vi "FlexMag - 23-03-2023.vi"() -> ()   [LabVIEW 2018] (continued)
                            }
                          }
                          n8986 = local read "CH3_Trns_BP_Right_DI"() -> (w14489:bool)
                          n8987 = case shown="False" w14489 {
                            tunnel: [FALSE ("CH1_Trns_BP_Left_DO") TRUE ("CH1_Trns_BP_Left_DO")] -> w14488
                            frame False {
                              n8988 = Wait Until Next ms Multiple(millisecond multiple=u32 200) -> ()  [unwired: 1 out]
                              n8989 = local write "CH3_Trns_BP_Right_DO"(TRUE ("CH1_Trns_BP_Left_DO")) -> ()
                            }
                            frame True {
                            }
                          }
                          n8990 = local read "ch2-3 transfer"() -> (w14496:bool)
                          n8991 = local read "ABORT"() -> (w14495:bool)
                          n8992 = Not(x=w14496) -> (.not. x?=w14494:bool)
                          n8993 = Compound Arithmetic op=OR(w14488, w14495, w14494) -> (w14493:bool)
                        }
                      }
                      frame True {
                      }
                    }
                  }
                }
              }
              frame #6 {
                n8994 = local read "ch2-3 transfer"() -> (w14503:bool)
                n8995 = case shown="True" w14503 {
                  frame False {
                  }
                  frame True {
                    n8996 = local read "ABORT"() -> (w14504:bool)
                    n8997 = case shown="False" w14504 {
                      frame False {
                        n8998 = local write "trns 2-3 led 2"(TRUE ("trns 1-2 led 1")) -> ()
                        n8999 = Wait (ms)(milliseconds to wait=u32 100) -> ()  [unwired: 1 out]
                      }
                      frame True {
                      }
                    }
                  }
                }
              }
              frame #7 {
                n9000 = local read "ch2-3 transfer"() -> (w14507:bool)
                n9001 = case shown="True" w14507 {
                  frame False {
                  }
                  frame True {
                    n9002 = local read "ABORT"() -> (w14508:bool)
                    n9003 = case shown="False" w14508 {
                      frame False {
                        n9004 = stacked-sequence {
                          frame #0 {
                            n9005 = local write "CH2_Trns_GV_Close_DO"(FALSE ("CH1_Trns_Gv_Close_DO")) -> ()
                            n9006 = Wait (ms)(milliseconds to wait=u32 100) -> ()  [unwired: 1 out]
                          }
                          frame #1 {
                            n9007 = while {
                              i -> [w14515]
                              stop <- w14516 stop-if-true
                              n9008 = Greater Or Equal?(x=w14515, y=600) -> (x >= y?=w14513:bool)
                              n9009 = case shown="True" w14513 {
                                frame False {
                                }
                                frame True {
                                n9010 = local write "trns error"(TRUE ("TRNS error")) -> ()
                                n9011 = local write "Warning Message"("Transfer process canceled!\nCH2-CH3 Trns GV couln't be opened" ("Warning Message")) -> ()
                                }
                              }
                              n9012 = local read "CH2_Trns_Gv_Open_DI"() -> (w14512:bool)
                              n9013 = case shown="False" w14512 {
                                tunnel: [FALSE ("CH1_Trns_BP_Left_DO") TRUE ("CH1_Trns_BP_Left_DO")] -> w14511
                                frame False {
                                n9014 = local write "CH2_Trns_GV_Open_DO"(TRUE ("CH1_Trns_BP_Left_DO")) -> ()
                                n9015 = Wait Until Next ms Multiple(millisecond multiple=u32 200) -> ()  [unwired: 1 out]
                                }
                                frame True {
                                }
                              }
                              n9016 = local read "ch2-3 transfer"() -> (w14519:bool)
                              n9017 = local read "ABORT"() -> (w14518:bool)
                              n9018 = Not(x=w14519) -> (.not. x?=w14517:bool)
                              n9019 = Compound Arithmetic op=OR(w14511, w14518, w14517) -> (w14516:bool)
                            }
                          }
                        }
                      }
                      frame True {
                      }
                    }
                  }
                }
              }
              frame #8 {
                n9020 = local read "ch2-3 transfer"() -> (w14526:bool)
                n9021 = case shown="True" w14526 {
                  frame False {
                  }
                  frame True {
                    n9022 = local read "ABORT"() -> (w14527:bool)
                    n9023 = case shown="False" w14527 {
                      frame False {
                        n9024 = local write "trns 2-3 led 3"(TRUE ("trns 1-2 led 1")) -> ()
                        n9025 = Wait (ms)(milliseconds to wait=u32 100) -> ()  [unwired: 1 out]
                      }
                      frame True {
                      }
                    }
                  }
                }
              }
              frame #9 {
                n9026 = local read "ch2-3 transfer"() -> (w14530:bool)
                n9027 = case shown="True" w14530 {
                  frame False {
                  }
                  frame True {
                    n9028 = local read "ABORT"() -> (w14531:bool)
                    n9029 = case shown="False" w14531 {
                      frame False {
                        n9030 = while {
                          i -> [w14536]
                          stop <- w14537 stop-if-true
                          n9031 = Greater Or Equal?(x=w14536, y=100) -> (x >= y?=w14534:bool)
                          n9032 = case shown="True" w14534 {
                            frame False {
                            }
                            frame True {
                              n9033 = local write "trns error"(TRUE ("TRNS error")) -> ()
                              n9034 = local write "Warning Message"("Transfer process canceled!\nCH2 TGV Control Problem" ("Warning Message")) -> ()
                            }
                          }
                          n9035 = local read "CH2_TGV_Control_DI"() -> (w14533:bool)
                          n9036 = case shown="True" w14533 {
                            tunnel: [TRUE ("CH1_Trns_BP_Left_DO") FALSE ("CH1_Trns_BP_Left_DO")] -> w14532
                            frame False {
                            }
                            frame True {
                              n9037 = Wait Until Next ms Multiple(millisecond multiple=u32 200) -> ()  [unwired: 1 out]
                              n9038 = local write "CH2_TGV_Control_DO"(FALSE ("CH1_Trns_BP_Left_DO")) -> ()
                            }
                          }
                          n9039 = local read "ch2-3 transfer"() -> (w14540:bool)
                          n9040 = local read "ABORT"() -> (w14539:bool)
                          n9041 = Not(x=w14540) -> (.not. x?=w14538:bool)
                          n9042 = Compound Arithmetic op=OR(w14532, w14539, w14538) -> (w14537:bool)
                        }
                      }
                      frame True {
                      }
                    }
                  }
                }
              }
              frame #10 {
                n9043 = local read "ch2-3 transfer"() -> (w14547:bool)
                n9044 = case shown="True" w14547 {
                  frame False {
                  }
                  frame True {
                    n9045 = local read "ABORT"() -> (w14548:bool)
                    n9046 = case shown="False" w14548 {
                      frame False {
                        n9047 = local write "trns 2-3 led 4"(TRUE ("trns 1-2 led 1")) -> ()
                        n9048 = Wait (ms)(milliseconds to wait=u32 100) -> ()  [unwired: 1 out]
                      }
                      frame True {
                      }
                    }
                  }
                }
              }
              frame #11 {
                n9049 = local read "ch2-3 transfer"() -> (w14551:bool)
                n9050 = case shown="True" w14551 {
                  frame False {
                  }
                  frame True {
                    n9051 = local read "ABORT"() -> (w14552:bool)
                    n9052 = case shown="False" w14552 {
                      frame False {
                        n9053 = while {
                          i -> [w14557]
                          stop <- w14558 stop-if-true
                          n9054 = local read "CH1_Trns_Interlock_DI"() -> (w14553:bool)
                          n9055 = Greater Or Equal?(x=w14557, y=100) -> (x >= y?=w14555:bool)
                          n9056 = case shown="True" w14555 {
                            frame False {
                            }
                            frame True {
                              n9057 = local write "Warning Message"("Transfer process canceled!\nCH1 Interlock problem" ("Warning Message")) -> ()
                              n9058 = local write "trns error"(TRUE ("TRNS error")) -> ()
                            }
                          }
                          n9059 = case shown="False" w14553 {
                            tunnel: [w14562 TRUE ("CH1_Trns_BP_Left_DO")] -> w14554
                            frame False {
                              n9060 = local read "CH1_TGV_Control_DI"() -> (w14563:bool)
                              n9061 = case shown="True" w14563 {
                                tunnel: [FALSE ("CH1_Trns_BP_Left_DO") TRUE ("CH1_Trns_BP_Left_DO")] -> w14562
                                frame False {
                                n9062 = Wait Until Next ms Multiple(millisecond multiple=u32 200) -> ()  [unwired: 1 out]
                                n9063 = local write "CH1_TGV_Control_DO"(TRUE ("CH1_Trns_BP_Left_DO")) -> ()
                                }
                                frame True {
                                }
                              }
                            }
                            frame True {
                            }
                          }
                          n9064 = local read "ch2-3 transfer"() -> (w14561:bool)
                          n9065 = local read "ABORT"() -> (w14560:bool)
                          n9066 = Not(x=w14561) -> (.not. x?=w14559:bool)
                          n9067 = Compound Arithmetic op=OR(w14554, w14560, w14559) -> (w14558:bool)
                        }
                      }
                      frame True {
                      }
                    }
                  }
                }
              }
              frame #12 {
                n9068 = local read "ch2-3 transfer"() -> (w14571:bool)
                n9069 = case shown="True" w14571 {
                  frame False {
                  }
                  frame True {
                    n9070 = local read "ABORT"() -> (w14572:bool)
                    n9071 = case shown="False" w14572 {
                      frame False {
                        w14573 = TRUE ("CH2_Right_Limit_DO")
                        n9072 = local write "trns 2-3 led 5"(TRUE ("trns 1-2 led 1")) -> ()
                        n9073 = Wait (ms)(milliseconds to wait=u32 100) -> ()  [unwired: 1 out]
                        n9074 = local write "CH2_Right_Limit_DO"(w14573) -> ()
                        n9075 = local write "CH2_Right_Slow_DO"(w14573) -> ()
                        n9076 = local write "CH2_Left_Slow_DO"(w14573) -> ()
                        n9077 = local write "CH2_Left_Limit_DO"(w14573) -> ()
                      }
                      frame True {
                      }
                    }
                  }
                }
              }
              frame #13 {
                n9078 = local read "ch2-3 transfer"() -> (w14576:bool)
                n9079 = case shown="True" w14576 {
                  frame False {
                  }
                  frame True {
                    n9080 = local read "ABORT"() -> (w14577:bool)
                    n9081 = case shown="False" w14577 {
                      frame False {
                        n9082 = while {
                          i -> [w14582]
                          stop <- w14583 stop-if-true
                          n9083 = local read "CH3_Trns_Interlock_DI"() -> (w14578:bool)
                          n9084 = Greater Or Equal?(x=w14582, y=100) -> (x >= y?=w14580:bool)
                          n9085 = case shown="True" w14580 {
                            frame False {
                            }
                            frame True {
                              n9086 = local write "Warning Message"("Transfer process canceled!\nCH3 Interlock problem" ("Warning Message")) -> ()
                              n9087 = local write "trns error"(TRUE ("TRNS error")) -> ()
                            }
                          }
                          n9088 = case shown="False" w14578 {
                            tunnel: [w14587 TRUE ("CH1_Trns_BP_Left_DO")] -> w14579
                            frame False {
                              n9089 = local read "CH3_TGV_Control_DI"() -> (w14588:bool)
                              n9090 = case shown="False" w14588 {
                                tunnel: [FALSE ("CH1_Trns_BP_Left_DO") TRUE ("CH1_Trns_BP_Left_DO")] -> w14587
                                frame False {
                                n9091 = Wait Until Next ms Multiple(millisecond multiple=u32 200) -> ()  [unwired: 1 out]
                                n9092 = local write "CH3_TGV_Control_DO"(TRUE ("CH1_Trns_BP_Left_DO")) -> ()
                                }
                                frame True {
                                }
                              }
                            }
                            frame True {
                            }
                          }
                          n9093 = local read "ch2-3 transfer"() -> (w14586:bool)
                          n9094 = local read "ABORT"() -> (w14585:bool)
                          n9095 = Not(x=w14586) -> (.not. x?=w14584:bool)
                          n9096 = Compound Arithmetic op=OR(w14579, w14585, w14584) -> (w14583:bool)
                        }
                      }
                      frame True {
                      }
                    }
                  }
                }
              }
              frame #14 {
                n9097 = local read "ch2-3 transfer"() -> (w14596:bool)
                n9098 = case shown="True" w14596 {
                  frame False {
                  }
                  frame True {
                    n9099 = local read "ABORT"() -> (w14597:bool)
                    n9100 = case shown="False" w14597 {
                      frame False {
                        n9101 = local write "trns 2-3 led 6"(TRUE ("trns 1-2 led 1")) -> ()
                        n9102 = Wait (ms)(milliseconds to wait=u32 100) -> ()  [unwired: 1 out]
                      }
                      frame True {
                      }
                    }
                  }
                }
              }
              frame #15 {
                n9103 = local read "ch2-3 transfer"() -> (w14600:bool)
                n9104 = case shown="True" w14600 {
                  frame False {
                  }
                  frame True {
                    n9105 = local read "ABORT"() -> (w14601:bool)
                    n9106 = case shown="False" w14601 {
                      frame False {
                        n9107 = while {
                          i -> [w14606]
                          stop <- w14607 stop-if-true
                          n9108 = local read "CH4_Trns_Interlock_DI"() -> (w14602:bool)
                          n9109 = Greater Or Equal?(x=w14606, y=100) -> (x >= y?=w14604:bool)
                          n9110 = case shown="True" w14604 {
                            frame False {
                            }
                            frame True {
                              n9111 = local write "Warning Message"("Transfer process canceled!\nCH4 Interlock problem" ("Warning Message")) -> ()
                              n9112 = local write "trns error"(TRUE ("TRNS error")) -> ()
                            }
                          }
                          n9113 = case shown="False" w14602 {
                            tunnel: [w14611 TRUE ("CH1_Trns_BP_Left_DO")] -> w14603
                            frame False {
                              n9114 = local read "CH4_TGV_Control_DI"() -> (w14612:bool)
                              n9115 = case shown="False" w14612 {
                                tunnel: [FALSE ("CH1_Trns_BP_Left_DO") TRUE ("CH1_Trns_BP_Left_DO")] -> w14611
                                frame False {
                                n9116 = Wait Until Next ms Multiple(millisecond multiple=u32 200) -> ()  [unwired: 1 out]
                                n9117 = local write "CH4_TGV_Control_DO"(TRUE ("CH1_Trns_BP_Left_DO")) -> ()
                                }
                                frame True {
                                }
                              }
                            }
                            frame True {
                            }
                          }
                          n9118 = local read "ch2-3 transfer"() -> (w14610:bool)
                          n9119 = local read "ABORT"() -> (w14609:bool)
                          n9120 = Not(x=w14610) -> (.not. x?=w14608:bool)
                          n9121 = Compound Arithmetic op=OR(w14603, w14609, w14608) -> (w14607:bool)
                        }
                      }
                      frame True {
                      }
                    }
                  }
                }
              }
              frame #16 {
                n9122 = local read "ch2-3 transfer"() -> (w14620:bool)
                n9123 = case shown="True" w14620 {
                  frame False {
                  }
                  frame True {
                    n9124 = local read "ABORT"() -> (w14621:bool)
                    n9125 = case shown="False" w14621 {
                      frame False {
                        n9126 = local write "trns 2-3 led 7"(TRUE ("trns 1-2 led 1")) -> ()
                        n9127 = Wait (ms)(milliseconds to wait=u32 100) -> ()  [unwired: 1 out]
                      }
                      frame True {
                      }
                    }
                  }
                }
              }
              frame #17 {
                n9128 = local read "ch2-3 transfer"() -> (w14624:bool)
                n9129 = case shown="True" w14624 {
                  frame False {
                  }
                  frame True {
                    n9130 = local read "ABORT"() -> (w14625:bool)
                    n9131 = case shown="False" w14625 {
                      frame False {
                        n9132 = while {
                          i -> [w14629]
                          stop <- w14630 stop-if-true
                          n9133 = Greater Or Equal?(x=w14629, y=100) -> (x >= y?=w14627:bool)
                          n9134 = case shown="True" w14627 {
                            frame False {
                            }
                            frame True {
                              n9135 = local write "Warning Message"("Transfer process canceled!\nRight Slow Sensor problem" ("Warning Message")) -> ()
                              n9136 = local write "trns error"(TRUE ("TRNS error")) -> ()
                            }
                          }
                          n9137 = disable-structure shown="Enabled" {
                            disable-tunnel: [w14635 w14640] -> w14626
                            frame Disabled {
                              n9138 = local read "Cnt_Right_Slow DI"() -> (w14634:bool)
                              n9139 = case shown="False" w14634 {
                                tunnel: [FALSE ("CH1_Trns_BP_Left_DO") TRUE ("CH1_Trns_BP_Left_DO")] -> w14635
                                frame False {
                                n9140 = Wait Until Next ms Multiple(millisecond multiple=u32 200) -> ()  [unwired: 1 out]
                                n9141 = local write "Cnt_Right_Slow DO"(TRUE ("CH1_Trns_BP_Left_DO")) -> ()
                                }
                                frame True {
                                }
                              }
                            }
                            frame Enabled {
                              n9142 = local read "CH2_Right_Slow_DI"() -> (w14641:bool)
                              n9143 = case shown="True" w14641 {
                                tunnel: [TRUE FALSE] -> w14640
                                frame False {
                                }
                                frame True {
                                n9144 = Wait Until Next ms Multiple(millisecond multiple=u32 200) -> ()  [unwired: 1 out]
                                n9145 = local write "CH2_Right_Slow_DO"(TRUE ("CH2_Right_Limit_DO")) -> ()
                                }
                              }
                            }
                          }
                          n9146 = local read "ch2-3 transfer"() -> (w14633:bool)
                          n9147 = local read "ABORT"() -> (w14632:bool)
                          n9148 = Not(x=w14633) -> (.not. x?=w14631:bool)
                          n9149 = Compound Arithmetic op=OR(w14626, w14632, w14631) -> (w14630:bool)
                        }
                      }
                      frame True {
                      }
                    }
                  }
                }
              }
              frame #18 {
                n9150 = local read "ch2-3 transfer"() -> (w14648:bool)
                n9151 = case shown="True" w14648 {
                  frame False {
                  }
                  frame True {
                    n9152 = local read "ABORT"() -> (w14649:bool)
                    n9153 = case shown="False" w14649 {
                      frame False {
                        n9154 = local write "trns 2-3 led 8"(TRUE ("trns 1-2 led 1")) -> ()
                        n9155 = Wait (ms)(milliseconds to wait=u32 100) -> ()  [unwired: 1 out]
                      }
                      frame True {
                      }
                    }
                  }
                }
              }
              frame #19 {
                n9156 = local read "ch2-3 transfer"() -> (w14652:bool)
                n9157 = case shown="True" w14652 {
                  frame False {
                  }
                  frame True {
                    n9158 = local read "ABORT"() -> (w14653:bool)
                    n9159 = case shown="False" w14653 {
                      frame False {
                        n9160 = while {
                          i -> [w14657]
                          stop <- w14658 stop-if-true
                          n9161 = Greater Or Equal?(x=w14657, y=100) -> (x >= y?=w14655:bool)
                          n9162 = case shown="True" w14655 {
                            frame False {
                            }
                            frame True {
                              n9163 = local write "Warning Message"("Transfer process canceled!\nRight Limit Sensor problem" ("Warning Message")) -> ()
                              n9164 = local write "trns error"(TRUE ("TRNS error")) -> ()
                            }
                          }
                          n9165 = disable-structure shown="Enabled" {
                            disable-tunnel: [w14663 w14668] -> w14654
                            frame Disabled {
                              n9166 = local read "Cnt_Right_Limit DI"() -> (w14662:bool)
                              n9167 = case shown="False" w14662 {
                                tunnel: [FALSE ("CH1_Trns_BP_Left_DO") TRUE ("CH1_Trns_BP_Left_DO")] -> w14663
                                frame False {
                                n9168 = Wait Until Next ms Multiple(millisecond multiple=u32 200) -> ()  [unwired: 1 out]
                                n9169 = local write "Cnt_Right_Limit DO"(TRUE ("CH1_Trns_BP_Left_DO")) -> ()
                                }
                                frame True {
                                }
                              }
                            }
                            frame Enabled {
                              n9170 = local read "CH2_Right_Limit_DI"() -> (w14669:bool)
                              n9171 = case shown="True" w14669 {
                                tunnel: [TRUE FALSE] -> w14668
                                frame False {
                                }
                                frame True {
                                n9172 = Wait Until Next ms Multiple(millisecond multiple=u32 200) -> ()  [unwired: 1 out]
                                n9173 = local write "CH2_Right_Limit_DO"(TRUE ("CH2_Right_Limit_DO")) -> ()
                                }
                              }
                            }
                          }
                          n9174 = local read "ch2-3 transfer"() -> (w14661:bool)
                          n9175 = local read "ABORT"() -> (w14660:bool)
                          n9176 = Not(x=w14661) -> (.not. x?=w14659:bool)
                          n9177 = Compound Arithmetic op=OR(w14654, w14660, w14659) -> (w14658:bool)
                        }
                      }
                      frame True {
                      }
                    }
                  }
                }
              }
              frame #20 {
                n9178 = local read "ch2-3 transfer"() -> (w14676:bool)
                n9179 = case shown="True" w14676 {
                  frame False {
                  }
                  frame True {
                    n9180 = local read "ABORT"() -> (w14677:bool)
                    n9181 = case shown="False" w14677 {
                      frame False {
                        n9182 = local write "trns 2-3 led 9"(TRUE ("trns 1-2 led 1")) -> ()
                        n9183 = Wait (ms)(milliseconds to wait=u32 100) -> ()  [unwired: 1 out]
                      }
                      frame True {
                      }
                    }
                  }
                }
              }
              frame #21 {
                n9184 = local read "ch2-3 transfer"() -> (w14680:bool)
                n9185 = case shown="True" w14680 {
                  frame False {
                  }
                  frame True {
                    n9186 = local read "ABORT"() -> (w14681:bool)
                    n9187 = case shown="False" w14681 {
                      frame False {
                        n9188 = while {
                          i -> [w14685]
                          stop <- w14686 stop-if-true
                          n9189 = Greater Or Equal?(x=w14685, y=100) -> (x >= y?=w14683:bool)
                          n9190 = case shown="True" w14683 {
                            frame False {
                            }
                            frame True {
                              n9191 = local write "Warning Message"("Transfer process canceled!\nLeft Slow Sensor problem" ("Warning Message")) -> ()
                              n9192 = local write "trns error"(TRUE ("TRNS error")) -> ()
                            }
                          }
                          n9193 = disable-structure shown="Enabled" {
                            disable-tunnel: [w14691 w14696] -> w14682
                            frame Disabled {
                              n9194 = local read "Cnt_Left_Slow DI"() -> (w14690:bool)
                              n9195 = case shown="False" w14690 {
                                tunnel: [FALSE ("CH1_Trns_BP_Left_DO") TRUE ("CH1_Trns_BP_Left_DO")] -> w14691
                                frame False {
                                n9196 = Wait Until Next ms Multiple(millisecond multiple=u32 200) -> ()  [unwired: 1 out]
                                n9197 = local write "Cnt_Left_Slow DO"(TRUE ("CH1_Trns_BP_Left_DO")) -> ()
                                }
                                frame True {
                                }
                              }
                            }
                            frame Enabled {
                              n9198 = local read "CH2_Left_Slow_DI"() -> (w14697:bool)
                              n9199 = case shown="True" w14697 {
                                tunnel: [TRUE FALSE] -> w14696
                                frame False {
                                }
                                frame True {
                                n9200 = Wait Until Next ms Multiple(millisecond multiple=u32 200) -> ()  [unwired: 1 out]
                                n9201 = local write "CH2_Left_Slow_DO"(TRUE ("CH2_Right_Limit_DO")) -> ()
                                }
                              }
                            }
                          }
                          n9202 = local read "ch2-3 transfer"() -> (w14689:bool)
                          n9203 = local read "ABORT"() -> (w14688:bool)
                          n9204 = Not(x=w14689) -> (.not. x?=w14687:bool)
                          n9205 = Compound Arithmetic op=OR(w14682, w14688, w14687) -> (w14686:bool)
                        }
                      }
                      frame True {
                      }
                    }
                  }
                }
              }
              frame #22 {
                n9206 = local read "ch2-3 transfer"() -> (w14704:bool)
                n9207 = case shown="True" w14704 {
                  frame False {
                  }
                  frame True {
                    n9208 = local read "ABORT"() -> (w14705:bool)
                    n9209 = case shown="False" w14705 {
                      frame False {
                        n9210 = local write "trns 2-3 led 10"(TRUE ("trns 1-2 led 1")) -> ()
                        n9211 = Wait (ms)(milliseconds to wait=u32 100) -> ()  [unwired: 1 out]
                      }
                      frame True {
                      }
                    }
                  }
                }
              }
              frame #23 {
                n9212 = local read "ch2-3 transfer"() -> (w14708:bool)
                n9213 = case shown="True" w14708 {
                  frame False {
                  }
                  frame True {
                    n9214 = local read "ABORT"() -> (w14709:bool)
                    n9215 = case shown="False" w14709 {
                      frame False {
                        n9216 = while {
                          i -> [w14713]
                          stop <- w14714 stop-if-true
                          n9217 = Greater Or Equal?(x=w14713, y=100) -> (x >= y?=w14711:bool)
                          n9218 = case shown="True" w14711 {
                            frame False {
                            }
                            frame True {
                              n9219 = local write "Warning Message"("Transfer process canceled!\nLeft Limit Sensor problem" ("Warning Message")) -> ()
                              n9220 = local write "trns error"(TRUE ("TRNS error")) -> ()
                            }
                          }
                          n9221 = disable-structure shown="Enabled" {
                            disable-tunnel: [w14719 w14724] -> w14710
                            frame Disabled {
                              n9222 = local read "Cnt_Left_Limit DI"() -> (w14718:bool)
                              n9223 = case shown="False" w14718 {
                                tunnel: [FALSE ("CH1_Trns_BP_Left_DO") TRUE ("CH1_Trns_BP_Left_DO")] -> w14719
                                frame False {
                                n9224 = Wait Until Next ms Multiple(millisecond multiple=u32 200) -> ()  [unwired: 1 out]
                                n9225 = local write "Cnt_Left_Limit DO"(TRUE ("CH1_Trns_BP_Left_DO")) -> ()
                                }
                                frame True {
                                }
                              }
                            }
                            frame Enabled {
                              n9226 = local read "CH2_Left_Limit_DI"() -> (w14725:bool)
                              n9227 = case shown="True" w14725 {
                                tunnel: [TRUE FALSE] -> w14724
                                frame False {
                                }
                                frame True {
                                n9228 = Wait Until Next ms Multiple(millisecond multiple=u32 200) -> ()  [unwired: 1 out]
                                n9229 = local write "CH2_Left_Limit_DO"(TRUE ("CH2_Right_Limit_DO")) -> ()
                                }
                              }
                            }
                          }
                          n9230 = local read "ch2-3 transfer"() -> (w14717:bool)
                          n9231 = local read "ABORT"() -> (w14716:bool)
                          n9232 = Not(x=w14717) -> (.not. x?=w14715:bool)
                          n9233 = Compound Arithmetic op=OR(w14710, w14716, w14715) -> (w14714:bool)
                        }
                      }
                      frame True {
                      }
                    }
                  }
                }
              }
              frame #24 {
                n9234 = local read "ch2-3 transfer"() -> (w14732:bool)
                n9235 = case shown="True" w14732 {
                  frame False {
                  }
                  frame True {
                    n9236 = local read "ABORT"() -> (w14733:bool)
                    n9237 = case shown="False" w14733 {
                      frame False {
                        n9238 = local write "trns 2-3 led 11"(TRUE ("trns 1-2 led 1")) -> ()
                        n9239 = Wait (ms)(milliseconds to wait=u32 100) -> ()  [unwired: 1 out]
                      }
                      frame True {
                      }
                    }
                  }
                }
              }
              frame #25 {
                n9240 = local read "ch2-3 transfer"() -> (w14736:bool)
                n9241 = case shown="True" w14736 {
                  frame False {
                  }
                  frame True {
                    n9242 = local read "ABORT"() -> (w14737:bool)
                    n9243 = case shown="False" w14737 {
                      frame False {
                        w14738 = FALSE ("CH4_SRV1_Piston_For_DO")
                        w14739 = TRUE ("CH4_SRV1_Piston_For_DO")
                        n9244 = local write "CH3_Right_Limit_DO"(w14739) -> ()
                        n9245 = local write "CH3_Right_Slow_DO"(w14739) -> ()
                        n9246 = local write "CH3_Left_Slow_DO"(w14738) -> ()
                        n9247 = local write "CH3_Left_Limit_DO"(w14738) -> ()
                        n9248 = Wait (ms)(milliseconds to wait=u32 2000) -> ()  [unwired: 1 out]
                      }
                      frame True {
                      }
                    }
                  }
                }
              }
              frame #26 {
                n9249 = local read "ch2-3 transfer"() -> (w14741:bool)
                n9250 = case shown="True" w14741 {
                  frame False {
                  }
                  frame True {
                    n9251 = local read "ABORT"() -> (w14742:bool)
                    n9252 = case shown="False" w14742 {
                      frame False {
                        n9253 = while {
                          i -> [w14747]
                          stop <- w14748 stop-if-true
                          n9254 = Greater Or Equal?(x=w14747, y=100) -> (x >= y?=w14745:bool)
                          n9255 = case shown="True" w14745 {
                            frame False {
                            }
                            frame True {
                              n9256 = local write "Warning Message"("Transfer process canceled!\nCassette Servo Direction problem" ("Warning Message")) -> ()
                              n9257 = local write "trns error"(TRUE ("TRNS error")) -> ()
                            }
                          }
                          n9258 = local read "Casette_Servo_Left_Direction DI"() -> (w14743:bool)
                          n9259 = case shown="False" w14743 {
                            tunnel: [FALSE ("CH1_Trns_BP_Left_DO") TRUE ("CH1_Trns_BP_Left_DO")] -> w14744
                            frame False {
                              n9260 = local write "Casette_Servo_Left_Direction DO"(TRUE ("CH1_Trns_BP_Left_DO")) -> ()
                              n9261 = Wait Until Next ms Multiple(millisecond multiple=u32 200) -> ()  [unwired: 1 out]
                            }
                            frame True {
                            }
                          }
                          n9262 = local read "ch2-3 transfer"() -> (w14751:bool)
                          n9263 = local read "ABORT"() -> (w14750:bool)
                          n9264 = Not(x=w14751) -> (.not. x?=w14749:bool)
                          n9265 = Compound Arithmetic op=OR(w14744, w14750, w14749) -> (w14748:bool)
                        }
                      }
                      frame True {
                      }
                    }
                  }
                }
              }
              frame #27 {
                n9266 = local read "ch2-3 transfer"() -> (w14758:bool)
                n9267 = case shown="True" w14758 {
                  frame False {
                  }
                  frame True {
                    n9268 = local read "ABORT"() -> (w14759:bool)
                    n9269 = case shown="False" w14759 {
                      frame False {
                        n9270 = local write "trns 2-3 led 12"(TRUE ("trns 1-2 led 1")) -> ()
                        n9271 = Wait (ms)(milliseconds to wait=u32 100) -> ()  [unwired: 1 out]
                      }
                      frame True {
                      }
                    }
                  }
                }
              }
              frame #28 {
                n9272 = local read "ch2-3 transfer"() -> (w14762:bool)
                n9273 = case shown="True" w14762 {
                  frame False {
                  }
                  frame True {
                    n9274 = local read "ABORT"() -> (w14763:bool)
                    n9275 = case shown="False" w14763 {
                      frame False {
                        n9276 = stacked-sequence {
                          frame #0 {
                            n9277 = local read "Cst_Speed_High"() -> (w14764:dbl)
                            n9278 = Wait (ms)(milliseconds to wait=u32 100) -> ()  [unwired: 1 out]
                            n9279 = local write "Cassette_Servo_Speed AO"(w14764) -> ()
                          }
                          frame #1 {
                            n9280 = Wait (ms)(milliseconds to wait=u32 200) -> ()  [unwired: 1 out]
                          }
                          frame #2 {
                            n9281 = local write "Cassette_Servo_Speed Set"(TRUE ("Cassette_Servo_Speed Set")) -> ()
                          }
                          frame #3 {
                            n9282 = Wait (ms)(milliseconds to wait=u32 300) -> ()  [unwired: 1 out]
                          }
                        }
                      }
                      frame True {
                      }
                    }
                  }
                }
              }
              frame #29 {
                n9283 = local read "ch2-3 transfer"() -> (w14769:bool)
                n9284 = case shown="True" w14769 {
                  frame False {
                  }
                  frame True {
                    n9285 = local read "ABORT"() -> (w14770:bool)
                    n9286 = case shown="False" w14770 {
                      frame False {
                        n9287 = local write "trns 2-3 led 13"(TRUE ("trns 1-2 led 1")) -> ()
                        n9288 = Wait (ms)(milliseconds to wait=u32 100) -> ()  [unwired: 1 out]
                      }
                      frame True {
                      }
                    }
                  }
                }
              }
              frame #30 {
                n9289 = local read "ch2-3 transfer"() -> (w14773:bool)
                n9290 = case shown="True" w14773 {
                  frame False {
                  }
                  frame True {
                    n9291 = local read "ABORT"() -> (w14774:bool)
                    n9292 = case shown="False" w14774 {
                      frame False {
                        n9293 = while {
                          i -> [w14779]
                          stop <- w14780 stop-if-true
                          n9294 = Greater Or Equal?(x=w14779, y=100) -> (x >= y?=w14777:bool)
                          n9295 = case shown="True" w14777 {
                            frame False {
                            }
                            frame True {
                              n9296 = local write "Warning Message"("Transfer process canceled!\nCassette Servo Start problem" ("Warning Message")) -> ()
                              n9297 = local write "trns error"(TRUE ("TRNS error")) -> ()
                            }
                          }
                          n9298 = local read "Casette_Servo_Start/Stop DI"() -> (w14775:bool)
                          n9299 = case shown="False" w14775 {
                            tunnel: [FALSE ("CH1_Trns_BP_Left_DO") TRUE ("CH1_Trns_BP_Left_DO")] -> w14776
                            frame False {
                              n9300 = local write "Casette_Servo_Start/Stop DO"(TRUE ("CH1_Trns_BP_Left_DO")) -> ()
                              n9301 = Wait Until Next ms Multiple(millisecond multiple=u32 200) -> ()  [unwired: 1 out]
                            }
                            frame True {
                            }
                          }
                          n9302 = local read "ch2-3 transfer"() -> (w14783:bool)
                          n9303 = local read "ABORT"() -> (w14782:bool)
                          n9304 = Not(x=w14783) -> (.not. x?=w14781:bool)
                          n9305 = Compound Arithmetic op=OR(w14776, w14782, w14781) -> (w14780:bool)
                        }
                      }
                      frame True {
                      }
                    }
                  }
                }
              }
              frame #31 {
                n9306 = local read "ch2-3 transfer"() -> (w14790:bool)
                n9307 = case shown="True" w14790 {
                  frame False {
                  }
                  frame True {
                    n9308 = local read "ABORT"() -> (w14791:bool)
                    n9309 = case shown="False" w14791 {
                      frame False {
                        n9310 = local write "trns 2-3 led 14"(TRUE ("trns 1-2 led 1")) -> ()
                        n9311 = Wait (ms)(milliseconds to wait=u32 100) -> ()  [unwired: 1 out]
                      }
                      frame True {
                      }
                    }
                  }
                }
              }
              frame #32 {
                n9312 = local read "ch2-3 transfer"() -> (w14794:bool)
                n9313 = case shown="True" w14794 {
                  frame False {
                  }
                  frame True {
                    n9314 = local read "ABORT"() -> (w14795:bool)
                    n9315 = case shown="False" w14795 {
                      frame False {
                        n9316 = disable-structure shown="Disabled" {
                          frame Disabled {
                            n9317 = stacked-sequence {
                              frame #0 {
                                n9318 = while {
                                i -> [w14802]
                                stop <- w14803 stop-if-true
                                n9319 = Greater Or Equal?(x=w14802, y=1500) -> (x >= y?=w14800:bool)
                                n9320 = case shown="True" w14800 {
                                frame False {
                                }
                                frame True {
                                n9321 = local write "Warning Message"("Transfer process canceled!\nCounter problem" ("Warning Message")) -> ()
                                n9322 = local write "trns error"(TRUE ("TRNS error")) -> ()
                                }
                                }
                                n9323 = local read "Counter Read Data"() -> (w14798:i16)
                                n9324 = Greater Or Equal?(x=w14798, y=i16 3686) -> (x >= y?=w14796:bool)
                                n9325 = case shown="True" w14796 {
                                tunnel: [FALSE ("CH1_Trns_BP_Left_DO") TRUE ("CH1_Trns_BP_Left_DO")] -> w14799
                                frame False {
                                n9326 = Wait Until Next ms Multiple(millisecond multiple=u32 200) -> ()  [unwired: 1 out]
                                }
                                frame True {
                                }
                                }
                                n9327 = local read "ch2-3 transfer"() -> (w14806:bool)
                                n9328 = local read "ABORT"() -> (w14805:bool)
                                n9329 = Not(x=w14806) -> (.not. x?=w14804:bool)
                                n9330 = Compound Arithmetic op=OR(w14799, w14805, w14804) -> (w14803:bool)
                                }
                              }
                              frame #1 {
                                n9331 = while {
                                i -> [w14816]
                                stop <- w14817 stop-if-true
                                n9332 = Greater Or Equal?(x=w14816, y=100) -> (x >= y?=w14814:bool)
                                n9333 = case shown="True" w14814 {
                                frame False {
                                }
                                frame True {
                                n9334 = local write "Warning Message"("Transfer process canceled!\nLeft Slow Sensor problem" ("Warning Message")) -> ()
                                n9335 = local write "trns error"(TRUE ("TRNS error")) -> ()
                                }
                                }
                                n9336 = local read "Cnt_Left_Slow DI"() -> (w14812:bool)
                                n9337 = case shown="True" w14812 {
                                tunnel: [TRUE ("CH1_Trns_BP_Left_DO") FALSE ("CH1_Trns_BP_Left_DO")] -> w14813
                                frame False {
                                }
                                frame True {
                                n9338 = local write "Cnt_Left_Slow DO"(FALSE ("TRNS error")) -> ()
                                n9339 = Wait Until Next ms Multiple(millisecond multiple=u32 200) -> ()  [unwired: 1 out]
                                }
                                }
                                n9340 = local read "ch2-3 transfer"() -> (w14820:bool)
                                n9341 = local read "ABORT"() -> (w14819:bool)
                                n9342 = Not(x=w14820) -> (.not. x?=w14818:bool)
                                n9343 = Compound Arithmetic op=OR(w14813, w14819, w14818) -> (w14817:bool)
                                }
                              }
                              frame #2 {
                                n9344 = while {
                                i -> [w14831]
                                stop <- w14832 stop-if-true
                                n9345 = Greater Or Equal?(x=w14831, y=100) -> (x >= y?=w14829:bool)
                                n9346 = case shown="True" w14829 {
                                frame False {
                                }
                                frame True {
                                n9347 = local write "Warning Message"("Transfer process canceled!\nLeft Limit Sensor problem" ("Warning Message")) -> ()
                                n9348 = local write "trns error"(TRUE ("TRNS error")) -> ()
                                }
                                }
                                n9349 = local read "Cnt_Left_Limit DI"() -> (w14827:bool)
                                n9350 = case shown="True" w14827 {
                                tunnel: [TRUE ("CH1_Trns_BP_Left_DO") FALSE ("CH1_Trns_BP_Left_DO")] -> w14828
                                frame False {
                                }
                                frame True {
                                n9351 = Wait Until Next ms Multiple(millisecond multiple=u32 200) -> ()  [unwired: 1 out]
                                n9352 = local write "Cnt_Left_Limit DO"(FALSE ("TRNS error")) -> ()
                                }
                                }
                                n9353 = local read "ch2-3 transfer"() -> (w14835:bool)
                                n9354 = local read "ABORT"() -> (w14834:bool)
                                n9355 = Not(x=w14835) -> (.not. x?=w14833:bool)
                                n9356 = Compound Arithmetic op=OR(w14828, w14834, w14833) -> (w14832:bool)
                                }
                              }
                            }
                          }
                          frame Enabled {
                          }
                        }
                      }
                      frame True {
                      }
                    }
                  }
                }
              }
              frame #33 {
                n9357 = local read "ch2-3 transfer"() -> (w14842:bool)
                n9358 = case shown="True" w14842 {
                  frame False {
                  }
                  frame True {
                    n9359 = local read "ABORT"() -> (w14843:bool)
                    n9360 = case shown="False" w14843 {
                      frame False {
                        n9361 = local write "trns 2-3 led 15"(TRUE ("trns 1-2 led 1")) -> ()
                        n9362 = Wait (ms)(milliseconds to wait=u32 100) -> ()  [unwired: 1 out]
                      }
                      frame True {
                      }
                    }
                  }
                }
              }
              frame #34 {
                n9363 = local read "ch2-3 transfer"() -> (w14846:bool)
                n9364 = case shown="True" w14846 {
                  frame False {
                  }
                  frame True {
                    n9365 = local read "ABORT"() -> (w14847:bool)
                    n9366 = case shown="False" w14847 {
                      frame False {
                        n9367 = stacked-sequence {
                          frame #0 {
                            n9368 = while {
                              i -> [w14852]
                              stop <- w14853 stop-if-true
                              n9369 = Greater Or Equal?(x=w14852, y=1500) -> (x >= y?=w14850:bool)
                              n9370 = case shown="True" w14850 {
                                frame False {
                                }
                                frame True {
                                n9371 = local write "Warning Message"("Transfer process canceled!\nCH3 Left Slow Sensor problem" ("Warning Message")) -> ()
                                n9372 = local write "trns error"(TRUE ("TRNS error")) -> ()
                                }
                              }
                              n9373 = local read "CH3_Left_Slow_DI"() -> (w14848:bool)
                              n9374 = case shown="False" w14848 {
                                tunnel: [FALSE ("CH1_Trns_BP_Left_DO") TRUE ("CH1_Trns_BP_Left_DO")] -> w14849
                                frame False {
                                n9375 = Wait Until Next ms Multiple(millisecond multiple=u32 200) -> ()  [unwired: 1 out]
                                }
                                frame True {
                                }
                              }
                              n9376 = local read "ch2-3 transfer"() -> (w14856:bool)
                              n9377 = local read "ABORT"() -> (w14855:bool)
                              n9378 = Not(x=w14856) -> (.not. x?=w14854:bool)
                              n9379 = Compound Arithmetic op=OR(w14849, w14855, w14854) -> (w14853:bool)
                            }
                          }
                          frame #1 {
                            n9380 = flat-sequence {
                              frame #0 {
                                n9381 = local read "Cst_Speed_Low"() -> (w14862:dbl)
                                n9382 = local write "Cassette_Servo_Speed AO"(w14862) -> ()
                                n9383 = Wait (ms)(milliseconds to wait=u32 100) -> ()  [unwired: 1 out]
                              }
                              frame #1 {
                                n9384 = local write "Cassette_Servo_Speed Set"(TRUE ("Cassette_Servo_Speed Set")) -> ()
                              }
                              frame #2 {
                                n9385 = Wait (ms)(milliseconds to wait=u32 100) -> ()  [unwired: 1 out]
                              }
                            }
                          }
                          frame #2 {
                            n9386 = while {
                              i -> [w14869]
                              stop <- w14870 stop-if-true
                              n9387 = Greater Or Equal?(x=w14869, y=100) -> (x >= y?=w14867:bool)
                              n9388 = case shown="True" w14867 {
                                frame False {
                                }
                                frame True {
                                n9389 = local write "Warning Message"("Transfer process canceled!\nLeft Slow Sensor problem" ("Warning Message")) -> ()
                                n9390 = local write "trns error"(TRUE ("TRNS error")) -> ()
                                }
                              }
                              n9391 = disable-structure shown="Enabled" {
                                disable-tunnel: [w14875 w14880] -> w14866
                                frame Disabled {
                                n9392 = local read "Cnt_Left_Slow DI"() -> (w14874:bool)
                                n9393 = case shown="False" w14874 {
                                tunnel: [FALSE ("CH1_Trns_BP_Left_DO") TRUE ("CH1_Trns_BP_Left_DO")] -> w14875
                                frame False {
                                n9394 = Wait Until Next ms Multiple(millisecond multiple=u32 200) -> ()  [unwired: 1 out]
                                n9395 = local write "Cnt_Left_Slow DO"(TRUE ("TRNS error")) -> ()
                                }
                                frame True {
                                }
                                }
                                }
                                frame Enabled {
                                n9396 = local read "CH3_Left_Slow_DI"() -> (w14881:bool)
                                n9397 = case shown="True" w14881 {
                                tunnel: [TRUE FALSE] -> w14880
                                frame False {
                                }
                                frame True {
                                n9398 = Wait Until Next ms Multiple(millisecond multiple=u32 200) -> ()  [unwired: 1 out]
                                n9399 = local write "CH3_Left_Slow_DO"(TRUE ("CH2_Right_Limit_DO")) -> ()
                                }
                                }
                                }
                              }
                              n9400 = local read "ch2-3 transfer"() -> (w14873:bool)